vi "FlexMag - 24-03-2023.vi"() -> ()   [LabVIEW 2018] (continued)
            n5541 = flat-sequence {
              frame #0 {
                n5542 = Wait (ms)(milliseconds to wait=u32 300) -> ()  [unwired: 1 out]
              }
              frame #1 {
                n5543 = local write "DC_auto_voltage_mode"(FALSE ("DC_auto_voltage_mode")) -> ()
              }
            }
            n5544 = VISA Write(VISA resource name=w10062, write buffer="\t\u0003\u0007\r", error in (no error)=w10061) -> (VISA resource name out=w10060:refnum<visa-resource-name>, error out=w10059:errorcluster)  [unwired: 1 out]
          }
        }
      }
    }
  }
  n5545 = while {
    tunnel: w77 -> [w10123]
    tunnel: w78 -> [w10122]
    tunnel: [w10121] -> w84
    tunnel: [w10120] -> w85
    tunnel: w80 -> [w10076]
    tunnel: w81 -> [w10075]
    tunnel: [w10074] -> w82
    tunnel: [w10073] -> w83
    stop <- FALSE stop-if-true
    # "According to manual, all starting addresses must be used increment"
    n5546 = Wait Until Next ms Multiple(millisecond multiple=u32 300) -> ()  [unwired: 1 out]
    n5547 = Or(x="TC1_set", y="TC1_auto_set") -> (x .or. y?=w10106:bool)
    n5548 = Or(x="TC2_set", y="TC2_auto_set") -> (x .or. y?=w10082:bool)
    n5549 = Build Array(FALSE, w10106, "TC1_open_loop_set", "TC1_close_loop_set", "TC1_P_set", "TC1_I_set", "TC1_D_set", "TC1_speed_gain_set", "TC1_speed_coefficient_set", "TC1_overspeed_set", "TC1_AO1_upper_limit_set", "TC1_AO1_bottom_limit_set", "TC1_AO1_polarity(neg_to_pos)", "TC1_AO1_polarity(pos_to_neg)", "TC1_display_tension_set", "TC1_display_AO1_set", "TC1_display_tension_actual", "TC1_display_AO1_actual", "TC1_tare_function", "TC1_regulation_type_selection", "TC1_setpoint_type", "TC1_reg_set") -> (w10126:bool[])
    n5550 = Build Array(FALSE, w10082, "TC2_open_loop_set", "TC2_close_loop_set", "TC2_P_set", "TC2_I_set", "TC2_D_set", "TC2_speed_gain_set", "TC2_speed_coefficient_set", "TC2_overspeed_set", "TC2_AO1_upper_limit_set", "TC2_AO1_bottom_limit_set", "TC2_AO1_polarity(neg_to_pos)", "TC2_AO1_polarity(pos_to_neg)", "TC2_display_tension_set", "TC2_display_AO1_set", "TC2_display_tension_actual", "TC2_display_AO1_actual", "TC2_tare_function", "TC2_regulation_type_selection", "TC2_setpoint_type", "TC2_reg_set") -> (w10099:bool[])
    n5551 = Boolean Array To Number(Boolean array=w10126) -> (number=w10127:u32)
    n5552 = Boolean Array To Number(Boolean array=w10099) -> (number=w10100:u32)
    n5553 = Mantissa & Exponent(0:w10127) -> (2:w10125:dbl)  [unwired: 1 out]
    n5554 = Mantissa & Exponent(0:w10100) -> (2:w10098:dbl)  [unwired: 1 out]
    n5555 = case shown="2" w10125 {
      tunnel: w10123 -> [w10689 w10699 w10721 w10743 w10765 w10787 w10809 w10831 w10853 w10875 w10897 w10919 w10941 w10963 w10985 w11007 w11029 w11051 w11073 w11097 w11116 w11135]
      tunnel: w10122 -> [w10688 w10698 w10720 w10742 w10764 w10786 w10808 w10830 w10852 w10874 w10896 w10918 w10940 w10962 w10984 w11006 w11028 w11050 w11072 w11096 w11115 w11134]
      tunnel: [w10687 w10702 w10724 w10746 w10768 w10790 w10812 w10834 w10856 w10878 w10900 w10922 w10944 w10966 w10988 w11010 w11032 w11054 w11075 w11081 w11100 w11120] -> w10121
      tunnel: [w10671 w10701 w10723 w10745 w10767 w10789 w10811 w10833 w10855 w10877 w10899 w10921 w10943 w10965 w10987 w11009 w11031 w11053 w11074 w11079 w11098 w11118] -> w10120
      frame 0, Default {
        # "this is important !\n9"
        n5556 = Increment(x=u16 294 ("Starting Address")) -> (x+1=w10685:u16)
        n5557 = call "MB Serial Master Query Read Holding Registers (poly).vi"("VISA resource name"=w10689, "Starting Address"=w10685, "Quantity"=u16 9, "error in"=w10688, "Serial Parameters"=T15 {"Mode"=enum."RTU", "Slave Address"=1}) -> ("VISA resource name out"=w10687:refnum<visa-resource-name>, "Holding Registers"=w10662:u16[], "error out"=w10671:errorcluster)  [unwired: 11 in, 1 out]
        n5558 = Index Array(array=w10662, index=0) -> (element=w10667:u16)
        n5559 = Index Array(array=w10662, index=2) -> (element=w10682:u16)
        n5560 = Index Array(array=w10662, index=4) -> (element=w10680:u16)
        n5561 = Index Array(array=w10662, index=8) -> (element=w10674:u16)
        n5562 = Index Array(array=w10662, index=6) -> (element=w10665:u16)
        n5563 = Type Cast(type=sgl 0.0, x=w10667) -> (*(type *) &x=w10633:sgl)
        n5564 = Type Cast(type=sgl 0.0, x=w10682) -> (*(type *) &x=w10670:sgl)
        "TC1_readout_set_value" <- w10670
        n5565 = Type Cast(type=sgl 0.0, x=w10680) -> (*(type *) &x=w10666:sgl)
        "TC1_measure_value" <- w10666
        n5566 = Type Cast(type=sgl 0.0, x=w10674) -> (*(type *) &x=w10642:sgl)
        n5567 = Type Cast(type=sgl 0.0, x=w10665) -> (*(type *) &x=→"TC1_diameter_readout":sgl)
        n5568 = Greater?(x=w10666, y=sgl 0.1) -> (0:w10677:bool)
        n5569 = Select(t=w10666, s=w10677, f=sgl 0.0) -> ()  [unwired: 1 out]
        n5570 = feedback #147() -> (w10660:sgl)  [unwired: 1 in]
        n5571 = feedback-in #147(w10670) -> ()
        n5572 = feedback #148() -> (w10636:sgl)  [unwired: 1 in]
        n5573 = feedback-in #148(w10633) -> ()
        n5574 = feedback #149() -> (w10658:sgl)  [unwired: 1 in]
        n5575 = feedback-in #149(w10660) -> ()
        n5576 = feedback #150() -> (w10637:sgl)  [unwired: 1 in]
        n5577 = feedback-in #150(w10636) -> ()
        n5578 = feedback #151() -> (w10657:sgl)  [unwired: 1 in]
        n5579 = feedback-in #151(w10658) -> ()
        n5580 = feedback #152() -> (w10645:sgl)  [unwired: 1 in]
        n5581 = feedback-in #152(w10642) -> ()
        n5582 = feedback #153() -> (w10638:sgl)  [unwired: 1 in]
        n5583 = feedback-in #153(w10637) -> ()
        n5584 = feedback #154() -> (w10656:sgl)  [unwired: 1 in]
        n5585 = feedback-in #154(w10657) -> ()
        n5586 = feedback #155() -> (w10639:sgl)  [unwired: 1 in]
        n5587 = feedback-in #155(w10638) -> ()
        n5588 = feedback #156() -> (w10646:sgl)  [unwired: 1 in]
        n5589 = feedback-in #156(w10645) -> ()
        n5590 = feedback #157() -> (w10655:sgl)  [unwired: 1 in]
        n5591 = feedback-in #157(w10656) -> ()
        n5592 = Compound Arithmetic op=ADD(w10633, w10636, w10637, w10638, w10639) -> (w10635:sgl)
        n5593 = feedback #158() -> (w10647:sgl)  [unwired: 1 in]
        n5594 = feedback-in #158(w10646) -> ()
        n5595 = feedback #159() -> (w10654:sgl)  [unwired: 1 in]
        n5596 = feedback-in #159(w10655) -> ()
        n5597 = feedback #160() -> (w10648:sgl)  [unwired: 1 in]
        n5598 = feedback-in #160(w10647) -> ()
        n5599 = Divide(x=w10635, y=5.0) -> (x/y=→"TC1_speed readout":dbl)
        n5600 = feedback #161() -> (w10653:sgl)  [unwired: 1 in]
        n5601 = feedback-in #161(w10654) -> ()
        n5602 = Compound Arithmetic op=ADD(w10642, w10645, w10646, w10647, w10648) -> (w10644:sgl)
        n5603 = feedback #162() -> (w10651:sgl)  [unwired: 1 in]
        n5604 = feedback-in #162(w10653) -> ()
        n5605 = Divide(x=w10644, y=5.0) -> (x/y=→"TC1_line speed readout":dbl)
        n5606 = feedback #163() -> (w10652:sgl)  [unwired: 1 in]
        n5607 = feedback-in #163(w10651) -> ()
        n5608 = Compound Arithmetic op=ADD(w10670, w10660, w10658, w10657, w10656, w10655, w10654, w10653, w10651, w10652) -> (w10659:sgl)
        n5609 = Divide(x=w10659, y=10.0) -> (x/y=→"TC1_Tension_read_set":dbl)
      }
      frame 1 {
        w10691 = FALSE ("TC1_set")
        w10700 = T15 {"Mode"=enum."RTU", "Slave Address"=1} ("Serial Parameters")
        n5610 = Type Cast(type=i16 0, x="TC1_set_value") -> (*(type *) &x=w10692:i16)
        n5611 = Build Array(w10692) -> (w10693:i16[])
        n5612 = Increment(x=u16 142) -> (x+1=w10697:u16)
        n5613 = call "MB Serial Master Query Write Multiple Registers (poly).vi"("VISA resource name"=w10699, "Starting Address"=w10697, "Registers"=w10693, "error in"=w10698, "Serial Parameters"=w10700) -> ("VISA resource name out"=w10707:refnum<visa-resource-name>, "error out"=w10706:errorcluster)  [unwired: 12 in, 1 out]
        n5614 = local write "TC1_auto_set"(w10691) -> ()
        n5615 = local write "TC1_set"(w10691) -> ()
        n5616 = Build Array(49152 ("element")) -> (w10705:i32[])
        n5617 = call "MB Serial Master Query Write Multiple Registers (poly).vi"("VISA resource name"=w10707, "Starting Address"=u16 320, "Registers"=w10705, "error in"=w10706, "Serial Parameters"=w10700) -> ("VISA resource name out"=w10711:refnum<visa-resource-name>, "error out"=w10712:errorcluster)  [unwired: 12 in, 1 out]
        n5618 = Build Array(49407 ("element")) -> (w10708:i32[])
        n5619 = call "MB Serial Master Query Write Multiple Registers (poly).vi"("VISA resource name"=w10711, "Starting Address"=u16 320, "Registers"=w10708, "error in"=w10712, "Serial Parameters"=w10700) -> ("VISA resource name out"=w10702:refnum<visa-resource-name>, "error out"=w10701:errorcluster)  [unwired: 12 in, 1 out]
      }
      frame 2 {
        w10722 = T15 {"Mode"=enum."RTU", "Slave Address"=1} ("Serial Parameters")
        n5620 = Type Cast(type=i16 0, x="TC1_open_loop_coefficient") -> (*(type *) &x=w10714:i16)
        n5621 = Build Array(w10714) -> (w10715:i16[])
        n5622 = Increment(x=u16 82) -> (x+1=w10719:u16)
        n5623 = call "MB Serial Master Query Write Multiple Registers (poly).vi"("VISA resource name"=w10721, "Starting Address"=w10719, "Registers"=w10715, "error in"=w10720, "Serial Parameters"=w10722) -> ("VISA resource name out"=w10729:refnum<visa-resource-name>, "error out"=w10728:errorcluster)  [unwired: 12 in, 1 out]
        n5624 = local write "TC1_open_loop_set"(FALSE ("TC1_open_loop_set")) -> ()
        n5625 = Build Array(49152 ("element")) -> (w10727:i32[])
        n5626 = call "MB Serial Master Query Write Multiple Registers (poly).vi"("VISA resource name"=w10729, "Starting Address"=u16 320, "Registers"=w10727, "error in"=w10728, "Serial Parameters"=w10722) -> ("VISA resource name out"=w10733:refnum<visa-resource-name>, "error out"=w10734:errorcluster)  [unwired: 12 in, 1 out]
        n5627 = Build Array(49407 ("element")) -> (w10730:i32[])
        n5628 = call "MB Serial Master Query Write Multiple Registers (poly).vi"("VISA resource name"=w10733, "Starting Address"=u16 320, "Registers"=w10730, "error in"=w10734, "Serial Parameters"=w10722) -> ("VISA resource name out"=w10724:refnum<visa-resource-name>, "error out"=w10723:errorcluster)  [unwired: 12 in, 1 out]
      }
      frame 3 {
        w10744 = T15 {"Mode"=enum."RTU", "Slave Address"=1} ("Serial Parameters")
        n5629 = Type Cast(type=i16 0, x="TC1_close_loop_coefficient") -> (*(type *) &x=w10736:i16)
        n5630 = Build Array(w10736) -> (w10737:i16[])
        n5631 = Increment(x=u16 84) -> (x+1=w10741:u16)
        n5632 = call "MB Serial Master Query Write Multiple Registers (poly).vi"("VISA resource name"=w10743, "Starting Address"=w10741, "Registers"=w10737, "error in"=w10742, "Serial Parameters"=w10744) -> ("VISA resource name out"=w10751:refnum<visa-resource-name>, "error out"=w10750:errorcluster)  [unwired: 12 in, 1 out]
        n5633 = local write "TC1_close_loop_set"(FALSE ("TC1_close_loop_set")) -> ()
        n5634 = Build Array(49152 ("element")) -> (w10749:i32[])
        n5635 = call "MB Serial Master Query Write Multiple Registers (poly).vi"("VISA resource name"=w10751, "Starting Address"=u16 320, "Registers"=w10749, "error in"=w10750, "Serial Parameters"=w10744) -> ("VISA resource name out"=w10755:refnum<visa-resource-name>, "error out"=w10756:errorcluster)  [unwired: 12 in, 1 out]
        n5636 = Build Array(49407 ("element")) -> (w10752:i32[])
        n5637 = call "MB Serial Master Query Write Multiple Registers (poly).vi"("VISA resource name"=w10755, "Starting Address"=u16 320, "Registers"=w10752, "error in"=w10756, "Serial Parameters"=w10744) -> ("VISA resource name out"=w10746:refnum<visa-resource-name>, "error out"=w10745:errorcluster)  [unwired: 12 in, 1 out]
      }
      frame 4 {
        w10766 = T15 {"Mode"=enum."RTU", "Slave Address"=1} ("Serial Parameters")
        n5638 = Type Cast(type=i16 0, x="TC1_P_coefficient") -> (*(type *) &x=w10758:i16)
        n5639 = Build Array(w10758) -> (w10759:i16[])
        n5640 = Increment(x=u16 108) -> (x+1=w10763:u16)
        n5641 = call "MB Serial Master Query Write Multiple Registers (poly).vi"("VISA resource name"=w10765, "Starting Address"=w10763, "Registers"=w10759, "error in"=w10764, "Serial Parameters"=w10766) -> ("VISA resource name out"=w10773:refnum<visa-resource-name>, "error out"=w10772:errorcluster)  [unwired: 12 in, 1 out]
        n5642 = local write "TC1_P_set"(FALSE ("TC1_P_set")) -> ()
        n5643 = Build Array(49152 ("element")) -> (w10771:i32[])
        n5644 = call "MB Serial Master Query Write Multiple Registers (poly).vi"("VISA resource name"=w10773, "Starting Address"=u16 320, "Registers"=w10771, "error in"=w10772, "Serial Parameters"=w10766) -> ("VISA resource name out"=w10777:refnum<visa-resource-name>, "error out"=w10778:errorcluster)  [unwired: 12 in, 1 out]
        n5645 = Build Array(49407 ("element")) -> (w10774:i32[])
        n5646 = call "MB Serial Master Query Write Multiple Registers (poly).vi"("VISA resource name"=w10777, "Starting Address"=u16 320, "Registers"=w10774, "error in"=w10778, "Serial Parameters"=w10766) -> ("VISA resource name out"=w10768:refnum<visa-resource-name>, "error out"=w10767:errorcluster)  [unwired: 12 in, 1 out]
      }
      frame 5 {
        w10788 = T15 {"Mode"=enum."RTU", "Slave Address"=1} ("Serial Parameters")
        n5647 = Type Cast(type=i16 0, x="TC1_I_coefficient") -> (*(type *) &x=w10780:i16)
        n5648 = Build Array(w10780) -> (w10781:i16[])
        n5649 = Increment(x=u16 110) -> (x+1=w10785:u16)
        n5650 = call "MB Serial Master Query Write Multiple Registers (poly).vi"("VISA resource name"=w10787, "Starting Address"=w10785, "Registers"=w10781, "error in"=w10786, "Serial Parameters"=w10788) -> ("VISA resource name out"=w10795:refnum<visa-resource-name>, "error out"=w10794:errorcluster)  [unwired: 12 in, 1 out]
        n5651 = local write "TC1_I_set"(FALSE ("TC1_I_set")) -> ()
        n5652 = Build Array(49152 ("element")) -> (w10793:i32[])
        n5653 = call "MB Serial Master Query Write Multiple Registers (poly).vi"("VISA resource name"=w10795, "Starting Address"=u16 320, "Registers"=w10793, "error in"=w10794, "Serial Parameters"=w10788) -> ("VISA resource name out"=w10799:refnum<visa-resource-name>, "error out"=w10800:errorcluster)  [unwired: 12 in, 1 out]
        n5654 = Build Array(49407 ("element")) -> (w10796:i32[])
        n5655 = call "MB Serial Master Query Write Multiple Registers (poly).vi"("VISA resource name"=w10799, "Starting Address"=u16 320, "Registers"=w10796, "error in"=w10800, "Serial Parameters"=w10788) -> ("VISA resource name out"=w10790:refnum<visa-resource-name>, "error out"=w10789:errorcluster)  [unwired: 12 in, 1 out]
      }
      frame 6 {
        w10810 = T15 {"Mode"=enum."RTU", "Slave Address"=1} ("Serial Parameters")
        n5656 = Type Cast(type=i16 0, x="TC1_D_coefficient") -> (*(type *) &x=w10802:i16)
        n5657 = Build Array(w10802) -> (w10803:i16[])
        n5658 = Increment(x=u16 112) -> (x+1=w10807:u16)
        n5659 = call "MB Serial Master Query Write Multiple Registers (poly).vi"("VISA resource name"=w10809, "Starting Address"=w10807, "Registers"=w10803, "error in"=w10808, "Serial Parameters"=w10810) -> ("VISA resource name out"=w10817:refnum<visa-resource-name>, "error out"=w10816:errorcluster)  [unwired: 12 in, 1 out]
        n5660 = local write "TC1_D_set"(FALSE ("TC1_D_set")) -> ()
        n5661 = Build Array(49152 ("element")) -> (w10815:i32[])
        n5662 = call "MB Serial Master Query Write Multiple Registers (poly).vi"("VISA resource name"=w10817, "Starting Address"=u16 320, "Registers"=w10815, "error in"=w10816, "Serial Parameters"=w10810) -> ("VISA resource name out"=w10821:refnum<visa-resource-name>, "error out"=w10822:errorcluster)  [unwired: 12 in, 1 out]
        n5663 = Build Array(49407 ("element")) -> (w10818:i32[])
        n5664 = call "MB Serial Master Query Write Multiple Registers (poly).vi"("VISA resource name"=w10821, "Starting Address"=u16 320, "Registers"=w10818, "error in"=w10822, "Serial Parameters"=w10810) -> ("VISA resource name out"=w10812:refnum<visa-resource-name>, "error out"=w10811:errorcluster)  [unwired: 12 in, 1 out]
      }
      frame 7 {
        w10832 = T15 {"Mode"=enum."RTU", "Slave Address"=1} ("Serial Parameters")
        n5665 = Type Cast(type=i16 0, x="TC1_speed_gain_value") -> (*(type *) &x=w10824:i16)
        n5666 = Build Array(w10824) -> (w10825:i16[])
        n5667 = Increment(x=u16 126) -> (x+1=w10829:u16)
        n5668 = call "MB Serial Master Query Write Multiple Registers (poly).vi"("VISA resource name"=w10831, "Starting Address"=w10829, "Registers"=w10825, "error in"=w10830, "Serial Parameters"=w10832) -> ("VISA resource name out"=w10839:refnum<visa-resource-name>, "error out"=w10838:errorcluster)  [unwired: 12 in, 1 out]
        n5669 = local write "TC1_speed_gain_set"(FALSE ("TC1_speed_gain_set")) -> ()
        n5670 = Build Array(49152 ("element")) -> (w10837:i32[])
        n5671 = call "MB Serial Master Query Write Multiple Registers (poly).vi"("VISA resource name"=w10839, "Starting Address"=u16 320, "Registers"=w10837, "error in"=w10838, "Serial Parameters"=w10832) -> ("VISA resource name out"=w10843:refnum<visa-resource-name>, "error out"=w10844:errorcluster)  [unwired: 12 in, 1 out]
        n5672 = Build Array(49407 ("element")) -> (w10840:i32[])
        n5673 = call "MB Serial Master Query Write Multiple Registers (poly).vi"("VISA resource name"=w10843, "Starting Address"=u16 320, "Registers"=w10840, "error in"=w10844, "Serial Parameters"=w10832) -> ("VISA resource name out"=w10834:refnum<visa-resource-name>, "error out"=w10833:errorcluster)  [unwired: 12 in, 1 out]
      }
      frame 8 {
        w10854 = T15 {"Mode"=enum."RTU", "Slave Address"=1} ("Serial Parameters")
        n5674 = Type Cast(type=i16 0, x="TC1_speed_coefficient_value") -> (*(type *) &x=w10846:i16)
        n5675 = Build Array(w10846) -> (w10847:i16[])
        n5676 = Increment(x=u16 128) -> (x+1=w10851:u16)
        n5677 = call "MB Serial Master Query Write Multiple Registers (poly).vi"("VISA resource name"=w10853, "Starting Address"=w10851, "Registers"=w10847, "error in"=w10852, "Serial Parameters"=w10854) -> ("VISA resource name out"=w10861:refnum<visa-resource-name>, "error out"=w10860:errorcluster)  [unwired: 12 in, 1 out]
        n5678 = local write "TC1_speed_coefficient_set"(FALSE ("TC1_speed_coefficient_set")) -> ()
        n5679 = Build Array(49152 ("element")) -> (w10859:i32[])
        n5680 = call "MB Serial Master Query Write Multiple Registers (poly).vi"("VISA resource name"=w10861, "Starting Address"=u16 320, "Registers"=w10859, "error in"=w10860, "Serial Parameters"=w10854) -> ("VISA resource name out"=w10865:refnum<visa-resource-name>, "error out"=w10866:errorcluster)  [unwired: 12 in, 1 out]
        n5681 = Build Array(49407 ("element")) -> (w10862:i32[])
        n5682 = call "MB Serial Master Query Write Multiple Registers (poly).vi"("VISA resource name"=w10865, "Starting Address"=u16 320, "Registers"=w10862, "error in"=w10866, "Serial Parameters"=w10854) -> ("VISA resource name out"=w10856:refnum<visa-resource-name>, "error out"=w10855:errorcluster)  [unwired: 12 in, 1 out]
      }
      frame 9 {
        w10876 = T15 {"Mode"=enum."RTU", "Slave Address"=1} ("Serial Parameters")
        n5683 = Type Cast(type=i16 0, x="TC1_overspeed_value") -> (*(type *) &x=w10868:i16)
        n5684 = Build Array(w10868) -> (w10869:i16[])
        n5685 = Increment(x=u16 130) -> (x+1=w10873:u16)
        n5686 = call "MB Serial Master Query Write Multiple Registers (poly).vi"("VISA resource name"=w10875, "Starting Address"=w10873, "Registers"=w10869, "error in"=w10874, "Serial Parameters"=w10876) -> ("VISA resource name out"=w10883:refnum<visa-resource-name>, "error out"=w10882:errorcluster)  [unwired: 12 in, 1 out]
        n5687 = local write "TC1_overspeed_set"(FALSE ("TC1_overspeed_set")) -> ()
        n5688 = Build Array(49152 ("element")) -> (w10881:i32[])
        n5689 = call "MB Serial Master Query Write Multiple Registers (poly).vi"("VISA resource name"=w10883, "Starting Address"=u16 320, "Registers"=w10881, "error in"=w10882, "Serial Parameters"=w10876) -> ("VISA resource name out"=w10887:refnum<visa-resource-name>, "error out"=w10888:errorcluster)  [unwired: 12 in, 1 out]
        n5690 = Build Array(49407 ("element")) -> (w10884:i32[])
        n5691 = call "MB Serial Master Query Write Multiple Registers (poly).vi"("VISA resource name"=w10887, "Starting Address"=u16 320, "Registers"=w10884, "error in"=w10888, "Serial Parameters"=w10876) -> ("VISA resource name out"=w10878:refnum<visa-resource-name>, "error out"=w10877:errorcluster)  [unwired: 12 in, 1 out]
      }
      frame 10 {
        w10898 = T15 {"Mode"=enum."RTU", "Slave Address"=1} ("Serial Parameters")
        n5692 = Type Cast(type=i16 0, x="TC1_AO1_upper_limit_value") -> (*(type *) &x=w10890:i16)
        n5693 = Build Array(w10890) -> (w10891:i16[])
        n5694 = Increment(x=u16 168) -> (x+1=w10895:u16)
        n5695 = call "MB Serial Master Query Write Multiple Registers (poly).vi"("VISA resource name"=w10897, "Starting Address"=w10895, "Registers"=w10891, "error in"=w10896, "Serial Parameters"=w10898) -> ("VISA resource name out"=w10905:refnum<visa-resource-name>, "error out"=w10904:errorcluster)  [unwired: 12 in, 1 out]
        n5696 = local write "TC1_AO1_upper_limit_set"(FALSE ("TC1_AO1_upper_limit_set")) -> ()
        n5697 = Build Array(49152 ("element")) -> (w10903:i32[])
        n5698 = call "MB Serial Master Query Write Multiple Registers (poly).vi"("VISA resource name"=w10905, "Starting Address"=u16 320, "Registers"=w10903, "error in"=w10904, "Serial Parameters"=w10898) -> ("VISA resource name out"=w10909:refnum<visa-resource-name>, "error out"=w10910:errorcluster)  [unwired: 12 in, 1 out]
        n5699 = Build Array(49407 ("element")) -> (w10906:i32[])
        n5700 = call "MB Serial Master Query Write Multiple Registers (poly).vi"("VISA resource name"=w10909, "Starting Address"=u16 320, "Registers"=w10906, "error in"=w10910, "Serial Parameters"=w10898) -> ("VISA resource name out"=w10900:refnum<visa-resource-name>, "error out"=w10899:errorcluster)  [unwired: 12 in, 1 out]
      }
      frame 11 {
        w10920 = T15 {"Mode"=enum."RTU", "Slave Address"=1} ("Serial Parameters")
        n5701 = Type Cast(type=i16 0, x="TC1_AO1_bottom_limit_value") -> (*(type *) &x=w10912:i16)
        n5702 = Build Array(w10912) -> (w10913:i16[])
        n5703 = Increment(x=u16 166) -> (x+1=w10917:u16)
        n5704 = call "MB Serial Master Query Write Multiple Registers (poly).vi"("VISA resource name"=w10919, "Starting Address"=w10917, "Registers"=w10913, "error in"=w10918, "Serial Parameters"=w10920) -> ("VISA resource name out"=w10927:refnum<visa-resource-name>, "error out"=w10926:errorcluster)  [unwired: 12 in, 1 out]
        n5705 = local write "TC1_AO1_bottom_limit_set"(FALSE ("TC1_AO1_bottom_limit_set")) -> ()
        n5706 = Build Array(49152 ("element")) -> (w10925:i32[])
        n5707 = call "MB Serial Master Query Write Multiple Registers (poly).vi"("VISA resource name"=w10927, "Starting Address"=u16 320, "Registers"=w10925, "error in"=w10926, "Serial Parameters"=w10920) -> ("VISA resource name out"=w10931:refnum<visa-resource-name>, "error out"=w10932:errorcluster)  [unwired: 12 in, 1 out]
        n5708 = Build Array(49407 ("element")) -> (w10928:i32[])
        n5709 = call "MB Serial Master Query Write Multiple Registers (poly).vi"("VISA resource name"=w10931, "Starting Address"=u16 320, "Registers"=w10928, "error in"=w10932, "Serial Parameters"=w10920) -> ("VISA resource name out"=w10922:refnum<visa-resource-name>, "error out"=w10921:errorcluster)  [unwired: 12 in, 1 out]
      }
      frame 12 {
        w10942 = T15 {"Mode"=enum."RTU", "Slave Address"=1} ("Serial Parameters")
        n5710 = Type Cast(type=i16 0, x=sgl 0.0 ("TC1_AO1_bottom_limit_value 2")) -> (*(type *) &x=w10934:i16)
        n5711 = Build Array(w10934) -> (w10935:i16[])
        n5712 = Increment(x=u16 198) -> (x+1=w10939:u16)
        n5713 = call "MB Serial Master Query Write Multiple Registers (poly).vi"("VISA resource name"=w10941, "Starting Address"=w10939, "Registers"=w10935, "error in"=w10940, "Serial Parameters"=w10942) -> ("VISA resource name out"=w10949:refnum<visa-resource-name>, "error out"=w10948:errorcluster)  [unwired: 12 in, 1 out]
        n5714 = local write "TC1_AO1_polarity(neg_to_pos)"(FALSE ("TC1_AO1_polarity(neg_to_pos)")) -> ()
        n5715 = Build Array(49152 ("element")) -> (w10947:i32[])
        n5716 = call "MB Serial Master Query Write Multiple Registers (poly).vi"("VISA resource name"=w10949, "Starting Address"=u16 320, "Registers"=w10947, "error in"=w10948, "Serial Parameters"=w10942) -> ("VISA resource name out"=w10953:refnum<visa-resource-name>, "error out"=w10954:errorcluster)  [unwired: 12 in, 1 out]
        n5717 = Build Array(49407 ("element")) -> (w10950:i32[])
        n5718 = call "MB Serial Master Query Write Multiple Registers (poly).vi"("VISA resource name"=w10953, "Starting Address"=u16 320, "Registers"=w10950, "error in"=w10954, "Serial Parameters"=w10942) -> ("VISA resource name out"=w10944:refnum<visa-resource-name>, "error out"=w10943:errorcluster)  [unwired: 12 in, 1 out]
      }
      frame 13 {
        w10964 = T15 {"Mode"=enum."RTU", "Slave Address"=1} ("Serial Parameters")
        n5719 = Type Cast(type=i16 0, x=sgl 1.0 ("TC1_AO1_bottom_limit_value 2")) -> (*(type *) &x=w10956:i16)
        n5720 = Build Array(w10956) -> (w10957:i16[])
        n5721 = Increment(x=u16 198) -> (x+1=w10961:u16)
        n5722 = call "MB Serial Master Query Write Multiple Registers (poly).vi"("VISA resource name"=w10963, "Starting Address"=w10961, "Registers"=w10957, "error in"=w10962, "Serial Parameters"=w10964) -> ("VISA resource name out"=w10971:refnum<visa-resource-name>, "error out"=w10970:errorcluster)  [unwired: 12 in, 1 out]
        n5723 = local write "TC1_AO1_polarity(pos_to_neg)"(FALSE ("TC1_AO1_polarity(pos_to_neg)")) -> ()
        n5724 = Build Array(49152 ("element")) -> (w10969:i32[])
        n5725 = call "MB Serial Master Query Write Multiple Registers (poly).vi"("VISA resource name"=w10971, "Starting Address"=u16 320, "Registers"=w10969, "error in"=w10970, "Serial Parameters"=w10964) -> ("VISA resource name out"=w10975:refnum<visa-resource-name>, "error out"=w10976:errorcluster)  [unwired: 12 in, 1 out]
        n5726 = Build Array(49407 ("element")) -> (w10972:i32[])
        n5727 = call "MB Serial Master Query Write Multiple Registers (poly).vi"("VISA resource name"=w10975, "Starting Address"=u16 320, "Registers"=w10972, "error in"=w10976, "Serial Parameters"=w10964) -> ("VISA resource name out"=w10966:refnum<visa-resource-name>, "error out"=w10965:errorcluster)  [unwired: 12 in, 1 out]
      }
      frame 14 {
        w10986 = T15 {"Mode"=enum."RTU", "Slave Address"=1} ("Serial Parameters")
        n5728 = Type Cast(type=i16 0, x=sgl 2.0 ("TC1_AO1_bottom_limit_value 2")) -> (*(type *) &x=w10978:i16)
        n5729 = Build Array(w10978) -> (w10979:i16[])
        n5730 = Increment(x=u16 8) -> (x+1=w10983:u16)
        n5731 = call "MB Serial Master Query Write Multiple Registers (poly).vi"("VISA resource name"=w10985, "Starting Address"=w10983, "Registers"=w10979, "error in"=w10984, "Serial Parameters"=w10986) -> ("VISA resource name out"=w10993:refnum<visa-resource-name>, "error out"=w10992:errorcluster)  [unwired: 12 in, 1 out]
        n5732 = local write "TC1_display_tension_set"(FALSE ("TC1_display_tension")) -> ()
        n5733 = Build Array(49152 ("element")) -> (w10991:i32[])
        n5734 = call "MB Serial Master Query Write Multiple Registers (poly).vi"("VISA resource name"=w10993, "Starting Address"=u16 320, "Registers"=w10991, "error in"=w10992, "Serial Parameters"=w10986) -> ("VISA resource name out"=w10997:refnum<visa-resource-name>, "error out"=w10998:errorcluster)  [unwired: 12 in, 1 out]
        n5735 = Build Array(49407 ("element")) -> (w10994:i32[])
        n5736 = call "MB Serial Master Query Write Multiple Registers (poly).vi"("VISA resource name"=w10997, "Starting Address"=u16 320, "Registers"=w10994, "error in"=w10998, "Serial Parameters"=w10986) -> ("VISA resource name out"=w10988:refnum<visa-resource-name>, "error out"=w10987:errorcluster)  [unwired: 12 in, 1 out]
      }
      frame 15 {
        w11008 = T15 {"Mode"=enum."RTU", "Slave Address"=1} ("Serial Parameters")
        n5737 = Type Cast(type=i16 0, x=sgl 5.0 ("TC1_AO1_bottom_limit_value 2")) -> (*(type *) &x=w11000:i16)
        n5738 = Build Array(w11000) -> (w11001:i16[])
        n5739 = Increment(x=u16 8) -> (x+1=w11005:u16)
        n5740 = call "MB Serial Master Query Write Multiple Registers (poly).vi"("VISA resource name"=w11007, "Starting Address"=w11005, "Registers"=w11001, "error in"=w11006, "Serial Parameters"=w11008) -> ("VISA resource name out"=w11015:refnum<visa-resource-name>, "error out"=w11014:errorcluster)  [unwired: 12 in, 1 out]
        n5741 = local write "TC1_display_AO1_set"(FALSE ("TC1_display_AO1")) -> ()
        n5742 = Build Array(49152 ("element")) -> (w11013:i32[])
        n5743 = call "MB Serial Master Query Write Multiple Registers (poly).vi"("VISA resource name"=w11015, "Starting Address"=u16 320, "Registers"=w11013, "error in"=w11014, "Serial Parameters"=w11008) -> ("VISA resource name out"=w11019:refnum<visa-resource-name>, "error out"=w11020:errorcluster)  [unwired: 12 in, 1 out]
        n5744 = Build Array(49407 ("element")) -> (w11016:i32[])
        n5745 = call "MB Serial Master Query Write Multiple Registers (poly).vi"("VISA resource name"=w11019, "Starting Address"=u16 320, "Registers"=w11016, "error in"=w11020, "Serial Parameters"=w11008) -> ("VISA resource name out"=w11010:refnum<visa-resource-name>, "error out"=w11009:errorcluster)  [unwired: 12 in, 1 out]
      }
      frame 16 {
        w11030 = T15 {"Mode"=enum."RTU", "Slave Address"=1} ("Serial Parameters")
        n5746 = Type Cast(type=i16 0, x=sgl 4.0 ("TC1_AO1_bottom_limit_value 2")) -> (*(type *) &x=w11022:i16)
        n5747 = Build Array(w11022) -> (w11023:i16[])
        n5748 = Increment(x=u16 10) -> (x+1=w11027:u16)
        n5749 = call "MB Serial Master Query Write Multiple Registers (poly).vi"("VISA resource name"=w11029, "Starting Address"=w11027, "Registers"=w11023, "error in"=w11028, "Serial Parameters"=w11030) -> ("VISA resource name out"=w11037:refnum<visa-resource-name>, "error out"=w11036:errorcluster)  [unwired: 12 in, 1 out]
        n5750 = local write "TC1_display_tension_actual"(FALSE ("TC1_display_tension")) -> ()
        n5751 = Build Array(49152 ("element")) -> (w11035:i32[])
        n5752 = call "MB Serial Master Query Write Multiple Registers (poly).vi"("VISA resource name"=w11037, "Starting Address"=u16 320, "Registers"=w11035, "error in"=w11036, "Serial Parameters"=w11030) -> ("VISA resource name out"=w11041:refnum<visa-resource-name>, "error out"=w11042:errorcluster)  [unwired: 12 in, 1 out]
        n5753 = Build Array(49407 ("element")) -> (w11038:i32[])
        n5754 = call "MB Serial Master Query Write Multiple Registers (poly).vi"("VISA resource name"=w11041, "Starting Address"=u16 320, "Registers"=w11038, "error in"=w11042, "Serial Parameters"=w11030) -> ("VISA resource name out"=w11032:refnum<visa-resource-name>, "error out"=w11031:errorcluster)  [unwired: 12 in, 1 out]
      }
      frame 17 {
        w11052 = T15 {"Mode"=enum."RTU", "Slave Address"=1} ("Serial Parameters")
        n5755 = Type Cast(type=i16 0, x=sgl 0.0 ("TC1_AO1_bottom_limit_value 2")) -> (*(type *) &x=w11044:i16)
        n5756 = Build Array(w11044) -> (w11045:i16[])
        n5757 = Increment(x=u16 10) -> (x+1=w11049:u16)
        n5758 = call "MB Serial Master Query Write Multiple Registers (poly).vi"("VISA resource name"=w11051, "Starting Address"=w11049, "Registers"=w11045, "error in"=w11050, "Serial Parameters"=w11052) -> ("VISA resource name out"=w11059:refnum<visa-resource-name>, "error out"=w11058:errorcluster)  [unwired: 12 in, 1 out]
        n5759 = local write "TC1_display_AO1_actual"(FALSE ("TC1_display_tension")) -> ()
        n5760 = Build Array(49152 ("element")) -> (w11057:i32[])
        n5761 = call "MB Serial Master Query Write Multiple Registers (poly).vi"("VISA resource name"=w11059, "Starting Address"=u16 320, "Registers"=w11057, "error in"=w11058, "Serial Parameters"=w11052) -> ("VISA resource name out"=w11063:refnum<visa-resource-name>, "error out"=w11064:errorcluster)  [unwired: 12 in, 1 out]
        n5762 = Build Array(49407 ("element")) -> (w11060:i32[])
        n5763 = call "MB Serial Master Query Write Multiple Registers (poly).vi"("VISA resource name"=w11063, "Starting Address"=u16 320, "Registers"=w11060, "error in"=w11064, "Serial Parameters"=w11052) -> ("VISA resource name out"=w11054:refnum<visa-resource-name>, "error out"=w11053:errorcluster)  [unwired: 12 in, 1 out]
      }
      frame 18 {
        n5764 = Build Array(u16 21767 ("Starting Address")) -> (w11067:u16[])
        n5765 = call "MB Serial Master Query Write Multiple Registers (poly).vi"("VISA resource name"=w11073, "Starting Address"=u16 322, "Registers"=w11067, "error in"=w11072, "Serial Parameters"=T15 {"Mode"=enum."RTU", "Slave Address"=1}) -> ("VISA resource name out"=w11069:refnum<visa-resource-name>, "error out"=w11068:errorcluster)  [unwired: 12 in, 1 out]
        n5766 = local write "TC1_tare_function"(FALSE ("TC1_tare_function")) -> ()
        n5767 = Build Array(49407 ("element")) -> (w11076:i32[])
        n5768 = call "MB Serial Master Query Write Multiple Registers (poly).vi"("VISA resource name"=w11069, "Starting Address"=u16 320, "Registers"=w11076, "error in"=w11068) -> ("VISA resource name out"=w11075:refnum<visa-resource-name>, "error out"=w11074:errorcluster)  [unwired: 13 in, 1 out]
      }
      frame 19 {
        w11080 = T15 {"Mode"=enum."RTU", "Slave Address"=1} ("Serial Parameters")
        n5769 = Build Array("TC1_regulation_type_value") -> (w11094:sgl[])
        n5770 = call "MB Serial Master Query Write Multiple Registers (poly).vi"("VISA resource name"=w11097, "Starting Address"=u16 107, "Registers"=w11094, "error in"=w11096, "Serial Parameters"=w11080) -> ("VISA resource name out"=w11083:refnum<visa-resource-name>, "error out"=w11082:errorcluster)  [unwired: 12 in, 1 out]
        n5771 = local write "TC1_regulation_type_selection"(FALSE ("TC1_tare_function")) -> ()
        n5772 = Build Array(49152 ("element")) -> (w11088:i32[])
        n5773 = call "MB Serial Master Query Write Multiple Registers (poly).vi"("VISA resource name"=w11083, "Starting Address"=u16 320, "Registers"=w11088, "error in"=w11082, "Serial Parameters"=w11080) -> ("VISA resource name out"=w11090:refnum<visa-resource-name>, "error out"=w11091:errorcluster)  [unwired: 12 in, 1 out]
        n5774 = Build Array(49407 ("element")) -> (w11089:i32[])
        n5775 = call "MB Serial Master Query Write Multiple Registers (poly).vi"("VISA resource name"=w11090, "Starting Address"=u16 320, "Registers"=w11089, "error in"=w11091, "Serial Parameters"=w11080) -> ("VISA resource name out"=w11081:refnum<visa-resource-name>, "error out"=w11079:errorcluster)  [unwired: 12 in, 1 out]
      }
      frame 20 {
        w11099 = T15 {"Mode"=enum."RTU", "Slave Address"=1} ("Serial Parameters")
        n5776 = Build Array("TC1_setpoint_type_value") -> (w11113:sgl[])
        n5777 = call "MB Serial Master Query Write Multiple Registers (poly).vi"("VISA resource name"=w11116, "Starting Address"=u16 141, "Registers"=w11113, "error in"=w11115, "Serial Parameters"=w11099) -> ("VISA resource name out"=w11102:refnum<visa-resource-name>, "error out"=w11101:errorcluster)  [unwired: 12 in, 1 out]
        n5778 = local write "TC1_setpoint_type"(FALSE ("TC1_tare_function")) -> ()
        n5779 = Build Array(49152 ("element")) -> (w11107:i32[])
        n5780 = call "MB Serial Master Query Write Multiple Registers (poly).vi"("VISA resource name"=w11102, "Starting Address"=u16 320, "Registers"=w11107, "error in"=w11101, "Serial Parameters"=w11099) -> ("VISA resource name out"=w11109:refnum<visa-resource-name>, "error out"=w11110:errorcluster)  [unwired: 12 in, 1 out]
        n5781 = Build Array(49407 ("element")) -> (w11108:i32[])
        n5782 = call "MB Serial Master Query Write Multiple Registers (poly).vi"("VISA resource name"=w11109, "Starting Address"=u16 320, "Registers"=w11108, "error in"=w11110, "Serial Parameters"=w11099) -> ("VISA resource name out"=w11100:refnum<visa-resource-name>, "error out"=w11098:errorcluster)  [unwired: 12 in, 1 out]
      }
      frame 21 {
        w11119 = T15 {"Mode"=enum."RTU", "Slave Address"=1} ("Serial Parameters")
        n5783 = Build Array("tc1 data set to reg") -> (w11133:sgl[])
        n5784 = call "MB Serial Master Query Write Multiple Registers (poly).vi"("VISA resource name"=w11135, "Starting Address"="tc1 Starting Address", "Registers"=w11133, "error in"=w11134, "Serial Parameters"=w11119) -> ("VISA resource name out"=w11122:refnum<visa-resource-name>, "error out"=w11121:errorcluster)  [unwired: 12 in, 1 out]
        n5785 = local write "TC1_reg_set"(FALSE ("TC1_tare_function")) -> ()
        n5786 = Build Array(49152 ("element")) -> (w11127:i32[])
        n5787 = call "MB Serial Master Query Write Multiple Registers (poly).vi"("VISA resource name"=w11122, "Starting Address"=u16 320, "Registers"=w11127, "error in"=w11121, "Serial Parameters"=w11119) -> ("VISA resource name out"=w11129:refnum<visa-resource-name>, "error out"=w11130:errorcluster)  [unwired: 12 in, 1 out]
        n5788 = Build Array(49407 ("element")) -> (w11128:i32[])
        n5789 = call "MB Serial Master Query Write Multiple Registers (poly).vi"("VISA resource name"=w11129, "Starting Address"=u16 320, "Registers"=w11128, "error in"=w11130, "Serial Parameters"=w11119) -> ("VISA resource name out"=w11120:refnum<visa-resource-name>, "error out"=w11118:errorcluster)  [unwired: 12 in, 1 out]
      }
    }
    n5790 = case shown="7" w10098 {
      tunnel: w10076 -> [w10186 w10196 w10218 w10240 w10262 w10284 w10306 w10328 w10350 w10372 w10394 w10416 w10438 w10460 w10482 w10504 w10526 w10548 w10570 w10580 w10599 w10619]
      tunnel: w10075 -> [w10185 w10195 w10217 w10239 w10261 w10283 w10305 w10321 w10349 w10371 w10393 w10415 w10437 w10459 w10481 w10503 w10525 w10547 w10569 w10579 w10598 w10618]
      tunnel: [w10184 w10199 w10221 w10243 w10265 w10287 w10309 w10331 w10353 w10375 w10397 w10419 w10441 w10463 w10485 w10507 w10529 w10551 w10572 w10581 w10600 w10620] -> w10074
      tunnel: [w10174 w10198 w10220 w10242 w10264 w10286 w10308 w10330 w10352 w10374 w10396 w10418 w10440 w10462 w10484 w10506 w10528 w10550 w10571 w10578 w10597 w10617] -> w10073
      frame 0, Default {
        n5791 = Increment(x=u16 294 ("Starting Address")) -> (x+1=w10182:u16)
        n5792 = call "MB Serial Master Query Read Holding Registers (poly).vi"("VISA resource name"=w10186, "Starting Address"=w10182, "Quantity"=u16 9, "error in"=w10185, "Serial Parameters"=T15 {"Mode"=enum."RTU", "Slave Address"=1}) -> ("VISA resource name out"=w10184:refnum<visa-resource-name>, "Holding Registers"=w10159:u16[], "error out"=w10174:errorcluster)  [unwired: 11 in, 1 out]
        n5793 = Index Array(array=w10159, index=2) -> (element=w10179:u16)
        n5794 = Index Array(array=w10159, index=8) -> (element=w10168:u16)
        n5795 = Index Array(array=w10159, index=4) -> (element=w10177:u16)
        n5796 = Index Array(array=w10159, index=0) -> (element=w10164:u16)
        n5797 = Index Array(array=w10159, index=6) -> (element=w10161:u16)
        n5798 = Type Cast(type=sgl 0.0, x=w10164) -> (*(type *) &x=w10131:sgl)
        n5799 = Type Cast(type=sgl 0.0, x=w10179) -> (*(type *) &x=w10167:sgl)
        "TC2_reading_set_value" <- w10167
        n5800 = Type Cast(type=sgl 0.0, x=w10168) -> (*(type *) &x=w10140:sgl)
        n5801 = Type Cast(type=sgl 0.0, x=w10177) -> (*(type *) &x=w10158:sgl)
        "TC2_measure_value" <- w10158
        n5802 = Type Cast(type=sgl 0.0, x=w10161) -> (*(type *) &x=→"TC2_diameter_readout":sgl)
        n5803 = Greater?(x=w10158, y=sgl 0.1) -> (0:w10173:bool)
        n5804 = Select(t=w10158, s=w10173, f=sgl 0.0) -> ()  [unwired: 1 out]
        n5805 = feedback #164() -> (w10133:sgl)  [unwired: 1 in]
        n5806 = feedback-in #164(w10131) -> ()
        n5807 = feedback #165() -> (w10134:sgl)  [unwired: 1 in]
        n5808 = feedback-in #165(w10133) -> ()
        n5809 = feedback #166() -> (w10147:sgl)  [unwired: 1 in]
        n5810 = feedback-in #166(w10167) -> ()
        n5811 = feedback #167() -> (w10135:sgl)  [unwired: 1 in]
        n5812 = feedback-in #167(w10134) -> ()
        n5813 = feedback #168() -> (w10148:sgl)  [unwired: 1 in]
        n5814 = feedback-in #168(w10147) -> ()
        n5815 = feedback #169() -> (w10136:sgl)  [unwired: 1 in]
        n5816 = feedback-in #169(w10135) -> ()
        n5817 = feedback #170() -> (w10141:sgl)  [unwired: 1 in]
        n5818 = feedback-in #170(w10140) -> ()
        n5819 = feedback #171() -> (w10149:sgl)  [unwired: 1 in]
        n5820 = feedback-in #171(w10148) -> ()
        n5821 = Compound Arithmetic op=ADD(w10131, w10133, w10134, w10135, w10136) -> (w10132:sgl)
        n5822 = feedback #172() -> (w10142:sgl)  [unwired: 1 in]
        n5823 = feedback-in #172(w10141) -> ()
        n5824 = feedback #173() -> (w10150:sgl)  [unwired: 1 in]
        n5825 = feedback-in #173(w10149) -> ()
        n5826 = feedback #174() -> (w10143:sgl)  [unwired: 1 in]
        n5827 = feedback-in #174(w10142) -> ()
        n5828 = Divide(x=w10132, y=5.0) -> (x/y=→"TC2_speed readout":dbl)
        n5829 = feedback #175() -> (w10151:sgl)  [unwired: 1 in]
        n5830 = feedback-in #175(w10150) -> ()
        n5831 = feedback #176() -> (w10144:sgl)  [unwired: 1 in]
        n5832 = feedback-in #176(w10143) -> ()
        n5833 = feedback #177() -> (w10152:sgl)  [unwired: 1 in]
        n5834 = feedback-in #177(w10151) -> ()
        n5835 = Compound Arithmetic op=ADD(w10140, w10141, w10142, w10143, w10144) -> (w10138:sgl)
        n5836 = feedback #178() -> (w10153:sgl)  [unwired: 1 in]
        n5837 = feedback-in #178(w10152) -> ()
        n5838 = feedback #179() -> (w10155:sgl)  [unwired: 1 in]
        n5839 = feedback-in #179(w10153) -> ()
        n5840 = Divide(x=w10138, y=5.0) -> (x/y=→"TC2_line speed readout":dbl)
        n5841 = feedback #180() -> (w10154:sgl)  [unwired: 1 in]
        n5842 = feedback-in #180(w10155) -> ()
        n5843 = Compound Arithmetic op=ADD(w10167, w10147, w10148, w10149, w10150, w10151, w10152, w10153, w10155, w10154) -> (w10146:sgl)
        n5844 = Divide(x=w10146, y=10.0) -> (x/y=→"TC2_Tension_read_set":dbl)
      }
      frame 1 {
        w10188 = FALSE ("TC2_set")
        w10197 = T15 {"Mode"=enum."RTU", "Slave Address"=1} ("Serial Parameters")
        n5845 = Type Cast(type=i16 0, x="TC2_set_value") -> (*(type *) &x=w10189:i16)
        n5846 = Build Array(w10189) -> (w10190:i16[])
        n5847 = Increment(x=u16 142) -> (x+1=w10194:u16)
        n5848 = call "MB Serial Master Query Write Multiple Registers (poly).vi"("VISA resource name"=w10196, "Starting Address"=w10194, "Registers"=w10190, "error in"=w10195, "Serial Parameters"=w10197) -> ("VISA resource name out"=w10204:refnum<visa-resource-name>, "error out"=w10203:errorcluster)  [unwired: 12 in, 1 out]
        n5849 = local write "TC2_auto_set"(w10188) -> ()
        n5850 = local write "TC2_set"(w10188) -> ()
        n5851 = Build Array(49152 ("element")) -> (w10202:i32[])
        n5852 = call "MB Serial Master Query Write Multiple Registers (poly).vi"("VISA resource name"=w10204, "Starting Address"=u16 320, "Registers"=w10202, "error in"=w10203, "Serial Parameters"=w10197) -> ("VISA resource name out"=w10208:refnum<visa-resource-name>, "error out"=w10209:errorcluster)  [unwired: 12 in, 1 out]
        n5853 = Build Array(49407 ("element")) -> (w10205:i32[])
        n5854 = call "MB Serial Master Query Write Multiple Registers (poly).vi"("VISA resource name"=w10208, "Starting Address"=u16 320, "Registers"=w10205, "error in"=w10209, "Serial Parameters"=w10197) -> ("VISA resource name out"=w10199:refnum<visa-resource-name>, "error out"=w10198:errorcluster)  [unwired: 12 in, 1 out]
      }
      frame 2 {
        w10219 = T15 {"Mode"=enum."RTU", "Slave Address"=1} ("Serial Parameters")
        n5855 = Type Cast(type=i16 0, x="TC2_open_loop_coefficient") -> (*(type *) &x=w10211:i16)
        n5856 = Build Array(w10211) -> (w10212:i16[])
        n5857 = Increment(x=u16 82) -> (x+1=w10216:u16)
        n5858 = call "MB Serial Master Query Write Multiple Registers (poly).vi"("VISA resource name"=w10218, "Starting Address"=w10216, "Registers"=w10212, "error in"=w10217, "Serial Parameters"=w10219) -> ("VISA resource name out"=w10226:refnum<visa-resource-name>, "error out"=w10225:errorcluster)  [unwired: 12 in, 1 out]
        n5859 = local write "TC2_open_loop_set"(FALSE ("TC2_open_loop_set")) -> ()
        n5860 = Build Array(49152 ("element")) -> (w10224:i32[])
        n5861 = call "MB Serial Master Query Write Multiple Registers (poly).vi"("VISA resource name"=w10226, "Starting Address"=u16 320, "Registers"=w10224, "error in"=w10225, "Serial Parameters"=w10219) -> ("VISA resource name out"=w10230:refnum<visa-resource-name>, "error out"=w10231:errorcluster)  [unwired: 12 in, 1 out]
        n5862 = Build Array(49407 ("element")) -> (w10227:i32[])
        n5863 = call "MB Serial Master Query Write Multiple Registers (poly).vi"("VISA resource name"=w10230, "Starting Address"=u16 320, "Registers"=w10227, "error in"=w10231, "Serial Parameters"=w10219) -> ("VISA resource name out"=w10221:refnum<visa-resource-name>, "error out"=w10220:errorcluster)  [unwired: 12 in, 1 out]
      }
      frame 3 {
        w10241 = T15 {"Mode"=enum."RTU", "Slave Address"=1} ("Serial Parameters")
        n5864 = Type Cast(type=i16 0, x="TC2_close_loop_coefficient") -> (*(type *) &x=w10233:i16)
        n5865 = Build Array(w10233) -> (w10234:i16[])
        n5866 = Increment(x=u16 84) -> (x+1=w10238:u16)
        n5867 = local write "TC2_close_loop_set"(FALSE ("TC2_close_loop_set")) -> ()
        n5868 = call "MB Serial Master Query Write Multiple Registers (poly).vi"("VISA resource name"=w10240, "Starting Address"=w10238, "Registers"=w10234, "error in"=w10239, "Serial Parameters"=w10241) -> ("VISA resource name out"=w10248:refnum<visa-resource-name>, "error out"=w10247:errorcluster)  [unwired: 12 in, 1 out]
        n5869 = Build Array(49152 ("element")) -> (w10246:i32[])
        n5870 = call "MB Serial Master Query Write Multiple Registers (poly).vi"("VISA resource name"=w10248, "Starting Address"=u16 320, "Registers"=w10246, "error in"=w10247, "Serial Parameters"=w10241) -> ("VISA resource name out"=w10252:refnum<visa-resource-name>, "error out"=w10253:errorcluster)  [unwired: 12 in, 1 out]
        n5871 = Build Array(49407 ("element")) -> (w10249:i32[])
        n5872 = call "MB Serial Master Query Write Multiple Registers (poly).vi"("VISA resource name"=w10252, "Starting Address"=u16 320, "Registers"=w10249, "error in"=w10253, "Serial Parameters"=w10241) -> ("VISA resource name out"=w10243:refnum<visa-resource-name>, "error out"=w10242:errorcluster)  [unwired: 12 in, 1 out]
      }
      frame 4 {
        w10263 = T15 {"Mode"=enum."RTU", "Slave Address"=1} ("Serial Parameters")
        n5873 = Type Cast(type=i16 0, x="TC2_P_coefficient") -> (*(type *) &x=w10255:i16)
        n5874 = Build Array(w10255) -> (w10256:i16[])
        n5875 = Increment(x=u16 108) -> (x+1=w10260:u16)
        n5876 = call "MB Serial Master Query Write Multiple Registers (poly).vi"("VISA resource name"=w10262, "Starting Address"=w10260, "Registers"=w10256, "error in"=w10261, "Serial Parameters"=w10263) -> ("VISA resource name out"=w10270:refnum<visa-resource-name>, "error out"=w10269:errorcluster)  [unwired: 12 in, 1 out]
        n5877 = local write "TC2_P_set"(FALSE ("TC2_P_set")) -> ()
        n5878 = Build Array(49152 ("element")) -> (w10268:i32[])
        n5879 = call "MB Serial Master Query Write Multiple Registers (poly).vi"("VISA resource name"=w10270, "Starting Address"=u16 320, "Registers"=w10268, "error in"=w10269, "Serial Parameters"=w10263) -> ("VISA resource name out"=w10274:refnum<visa-resource-name>, "error out"=w10275:errorcluster)  [unwired: 12 in, 1 out]
        n5880 = Build Array(49407 ("element")) -> (w10271:i32[])
        n5881 = call "MB Serial Master Query Write Multiple Registers (poly).vi"("VISA resource name"=w10274, "Starting Address"=u16 320, "Registers"=w10271, "error in"=w10275, "Serial Parameters"=w10263) -> ("VISA resource name out"=w10265:refnum<visa-resource-name>, "error out"=w10264:errorcluster)  [unwired: 12 in, 1 out]
      }
      frame 5 {
        w10285 = T15 {"Mode"=enum."RTU", "Slave Address"=1} ("Serial Parameters")
        n5882 = Type Cast(type=i16 0, x="TC2_I_coefficient") -> (*(type *) &x=w10277:i16)
        n5883 = Build Array(w10277) -> (w10278:i16[])
        n5884 = Increment(x=u16 110) -> (x+1=w10282:u16)
        n5885 = call "MB Serial Master Query Write Multiple Registers (poly).vi"("VISA resource name"=w10284, "Starting Address"=w10282, "Registers"=w10278, "error in"=w10283, "Serial Parameters"=w10285) -> ("VISA resource name out"=w10292:refnum<visa-resource-name>, "error out"=w10291:errorcluster)  [unwired: 12 in, 1 out]
        n5886 = local write "TC2_I_set"(FALSE ("TC2_I_set")) -> ()
        n5887 = Build Array(49152 ("element")) -> (w10290:i32[])
        n5888 = call "MB Serial Master Query Write Multiple Registers (poly).vi"("VISA resource name"=w10292, "Starting Address"=u16 320, "Registers"=w10290, "error in"=w10291, "Serial Parameters"=w10285) -> ("VISA resource name out"=w10296:refnum<visa-resource-name>, "error out"=w10297:errorcluster)  [unwired: 12 in, 1 out]
        n5889 = Build Array(49407 ("element")) -> (w10293:i32[])
        n5890 = call "MB Serial Master Query Write Multiple Registers (poly).vi"("VISA resource name"=w10296, "Starting Address"=u16 320, "Registers"=w10293, "error in"=w10297, "Serial Parameters"=w10285) -> ("VISA resource name out"=w10287:refnum<visa-resource-name>, "error out"=w10286:errorcluster)  [unwired: 12 in, 1 out]
      }
      frame 6 {
        w10307 = T15 {"Mode"=enum."RTU", "Slave Address"=1} ("Serial Parameters")
        n5891 = Type Cast(type=i16 0, x="TC2_D_coefficient") -> (*(type *) &x=w10299:i16)
        n5892 = Build Array(w10299) -> (w10300:i16[])
        n5893 = Increment(x=u16 112) -> (x+1=w10304:u16)
        n5894 = call "MB Serial Master Query Write Multiple Registers (poly).vi"("VISA resource name"=w10306, "Starting Address"=w10304, "Registers"=w10300, "error in"=w10305, "Serial Parameters"=w10307) -> ("VISA resource name out"=w10314:refnum<visa-resource-name>, "error out"=w10313:errorcluster)  [unwired: 12 in, 1 out]
        n5895 = local write "TC2_D_set"(FALSE ("TC2_D_set")) -> ()
        n5896 = Build Array(49152 ("element")) -> (w10312:i32[])
        n5897 = call "MB Serial Master Query Write Multiple Registers (poly).vi"("VISA resource name"=w10314, "Starting Address"=u16 320, "Registers"=w10312, "error in"=w10313, "Serial Parameters"=w10307) -> ("VISA resource name out"=w10318:refnum<visa-resource-name>, "error out"=w10319:errorcluster)  [unwired: 12 in, 1 out]
        n5898 = Build Array(49407 ("element")) -> (w10315:i32[])
        n5899 = call "MB Serial Master Query Write Multiple Registers (poly).vi"("VISA resource name"=w10318, "Starting Address"=u16 320, "Registers"=w10315, "error in"=w10319, "Serial Parameters"=w10307) -> ("VISA resource name out"=w10309:refnum<visa-resource-name>, "error out"=w10308:errorcluster)  [unwired: 12 in, 1 out]
      }
      frame 7 {
        w10329 = T15 {"Mode"=enum."RTU", "Slave Address"=1} ("Serial Parameters")
        n5900 = Type Cast(type=i16 0, x="TC2_speed_gain_value") -> (*(type *) &x=w10322:i16)
        n5901 = Build Array(w10322) -> (w10323:i16[])
        n5902 = Increment(x=u16 126) -> (x+1=w10327:u16)
        n5903 = local write "TC2_speed_gain_set"(FALSE ("TC2_speed_gain_set")) -> ()
        n5904 = call "MB Serial Master Query Write Multiple Registers (poly).vi"("VISA resource name"=w10328, "Starting Address"=w10327, "Registers"=w10323, "error in"=w10321, "Serial Parameters"=w10329) -> ("VISA resource name out"=w10336:refnum<visa-resource-name>, "error out"=w10335:errorcluster)  [unwired: 12 in, 1 out]
        n5905 = Build Array(49152 ("element")) -> (w10334:i32[])
        n5906 = call "MB Serial Master Query Write Multiple Registers (poly).vi"("VISA resource name"=w10336, "Starting Address"=u16 320, "Registers"=w10334, "error in"=w10335, "Serial Parameters"=w10329) -> ("VISA resource name out"=w10340:refnum<visa-resource-name>, "error out"=w10341:errorcluster)  [unwired: 12 in, 1 out]
        n5907 = Build Array(49407 ("element")) -> (w10337:i32[])
        n5908 = call "MB Serial Master Query Write Multiple Registers (poly).vi"("VISA resource name"=w10340, "Starting Address"=u16 320, "Registers"=w10337, "error in"=w10341, "Serial Parameters"=w10329) -> ("VISA resource name out"=w10331:refnum<visa-resource-name>, "error out"=w10330:errorcluster)  [unwired: 12 in, 1 out]
      }
      frame 8 {
        w10351 = T15 {"Mode"=enum."RTU", "Slave Address"=1} ("Serial Parameters")
        n5909 = Type Cast(type=i16 0, x="TC2_speed_coefficient_value") -> (*(type *) &x=w10343:i16)
        n5910 = Build Array(w10343) -> (w10344:i16[])
        n5911 = Increment(x=u16 128) -> (x+1=w10348:u16)
        n5912 = call "MB Serial Master Query Write Multiple Registers (poly).vi"("VISA resource name"=w10350, "Starting Address"=w10348, "Registers"=w10344, "error in"=w10349, "Serial Parameters"=w10351) -> ("VISA resource name out"=w10358:refnum<visa-resource-name>, "error out"=w10357:errorcluster)  [unwired: 12 in, 1 out]
        n5913 = local write "TC2_speed_coefficient_set"(FALSE ("TC2_speed_coefficient_set")) -> ()
        n5914 = Build Array(49152 ("element")) -> (w10356:i32[])
        n5915 = call "MB Serial Master Query Write Multiple Registers (poly).vi"("VISA resource name"=w10358, "Starting Address"=u16 320, "Registers"=w10356, "error in"=w10357, "Serial Parameters"=w10351) -> ("VISA resource name out"=w10362:refnum<visa-resource-name>, "error out"=w10363:errorcluster)  [unwired: 12 in, 1 out]
        n5916 = Build Array(49407 ("element")) -> (w10359:i32[])
        n5917 = call "MB Serial Master Query Write Multiple Registers (poly).vi"("VISA resource name"=w10362, "Starting Address"=u16 320, "Registers"=w10359, "error in"=w10363, "Serial Parameters"=w10351) -> ("VISA resource name out"=w10353:refnum<visa-resource-name>, "error out"=w10352:errorcluster)  [unwired: 12 in, 1 out]
      }
      frame 9 {
        w10373 = T15 {"Mode"=enum."RTU", "Slave Address"=1} ("Serial Parameters")
        n5918 = Type Cast(type=i16 0, x="TC2_overspeed_value") -> (*(type *) &x=w10365:i16)
        n5919 = Build Array(w10365) -> (w10366:i16[])
        n5920 = Increment(x=u16 130) -> (x+1=w10370:u16)
        n5921 = call "MB Serial Master Query Write Multiple Registers (poly).vi"("VISA resource name"=w10372, "Starting Address"=w10370, "Registers"=w10366, "error in"=w10371, "Serial Parameters"=w10373) -> ("VISA resource name out"=w10380:refnum<visa-resource-name>, "error out"=w10379:errorcluster)  [unwired: 12 in, 1 out]
        n5922 = local write "TC2_overspeed_set"(FALSE ("TC2_overspeed_set")) -> ()
        n5923 = Build Array(49152 ("element")) -> (w10378:i32[])
        n5924 = call "MB Serial Master Query Write Multiple Registers (poly).vi"("VISA resource name"=w10380, "Starting Address"=u16 320, "Registers"=w10378, "error in"=w10379, "Serial Parameters"=w10373) -> ("VISA resource name out"=w10384:refnum<visa-resource-name>, "error out"=w10385:errorcluster)  [unwired: 12 in, 1 out]
        n5925 = Build Array(49407 ("element")) -> (w10381:i32[])
        n5926 = call "MB Serial Master Query Write Multiple Registers (poly).vi"("VISA resource name"=w10384, "Starting Address"=u16 320, "Registers"=w10381, "error in"=w10385, "Serial Parameters"=w10373) -> ("VISA resource name out"=w10375:refnum<visa-resource-name>, "error out"=w10374:errorcluster)  [unwired: 12 in, 1 out]
      }
      frame 10 {
        w10395 = T15 {"Mode"=enum."RTU", "Slave Address"=1} ("Serial Parameters")
        n5927 = Type Cast(type=i16 0, x="TC2_AO1_upper_limit_value") -> (*(type *) &x=w10387:i16)
        n5928 = Build Array(w10387) -> (w10388:i16[])
        n5929 = Increment(x=u16 168) -> (x+1=w10392:u16)
        n5930 = call "MB Serial Master Query Write Multiple Registers (poly).vi"("VISA resource name"=w10394, "Starting Address"=w10392, "Registers"=w10388, "error in"=w10393, "Serial Parameters"=w10395) -> ("VISA resource name out"=w10402:refnum<visa-resource-name>, "error out"=w10401:errorcluster)  [unwired: 12 in, 1 out]
        n5931 = local write "TC2_AO1_upper_limit_set"(FALSE ("TC2_AO1_upper_limit_set")) -> ()